vi "HFRR ADV v039.vi"() -> ()   [LabVIEW 2025] (continued)
                      }
                    }
                  }
                }
              }
            }
          }
          frame Enabled {
          }
        }
        n284 = Get Date/Time In Seconds() -> (seconds since 1Jan1904=w369:timestamp)
        n285 = Format Into String(format string="%<%I:%M:%S:%p %d:%B:%Y>T", w369) -> (resulting string=→"Time Stamp":string)  [unwired: 2 in, 1 out]
        n286 = local read "Service Password enable"() -> (w361:bool)
        n287 = local read "FILE"() -> (w366:string)
        n288 = call <vilib>:"Trim Whitespace.vi"("string"=w366) -> ("trimmed string"=w365:string)  [unwired: 1 in]
        n289 = String Length(string=w365) -> (length=w364:i32)
        n290 = Greater?(x=w364, y=1) -> (0:w362:bool)
        n291 = case shown="False" w362 {
          tunnel: w361 -> [w390 _]
          frame False {
            n292 = case shown="False" w390 {
              frame True {
                w391 = "Test Start In Service Mode" ("Tip Strip")
                w392 = T19."Enabled" ("Disabled")
                n293 = property on="Auto Start Test" class="Bool (strict)"("DisabledEnum"=w392, "TipStrip"=w391) -> ()  [unwired: 2 in, 2 out]
                n294 = property on="RUN" class="Bool (strict)"("DisabledEnum"=w392, "TipStrip"=w391) -> ()  [unwired: 2 in, 2 out]
              }
              frame False {
                w393 = "Enter File Name to Start Test" ("Tip Strip")
                w394 = T19."Disabled and Grayed Out" ("Disabled")
                n295 = property on="Auto Start Test" class="Bool (strict)"("DisabledEnum"=w394, "TipStrip"=w393) -> ()  [unwired: 2 in, 2 out]
                n296 = property on="RUN" class="Bool (strict)"("DisabledEnum"=w394, "TipStrip"=w393) -> ()  [unwired: 2 in, 2 out]
              }
            }
          }
          frame True {
            w395 = "" ("Tip Strip")
            w396 = T19."Enabled" ("Disabled")
            n297 = property on="Auto Start Test" class="Bool (strict)"("DisabledEnum"=w396, "TipStrip"=w395) -> ()  [unwired: 2 in, 2 out]
            n298 = property on="RUN" class="Bool (strict)"("DisabledEnum"=w396, "TipStrip"=w395) -> ()  [unwired: 2 in, 2 out]
          }
        }
      }
      event "RUN": Value Change {
        n299 = event-data() -> ()  [unwired: 1 in, 6 out]
        n300 = local read "RUN"() -> (w398:bool)
        n301 = case shown="False" w398 {
          frame False {
            n302 = flat-sequence {
              frame #0 {
                n303 = local write "START TEMP"(FALSE ("START TEMP")) -> ()
              }
              frame #1 {
                n304 = Wait (ms)(milliseconds to wait=u32 1500) -> ()  [unwired: 1 out]
              }
              frame #2 {
                n305 = local write "Humidity 2"(TRUE ("Humidity")) -> ()
              }
              frame #3 {
                n306 = local write "Due Write"("VC;0") -> ()
              }
              frame #4 {
                n307 = Wait (ms)(milliseconds to wait=u32 1500) -> ()  [unwired: 1 out]
              }
              frame #5 {
                w408 = T19."Enabled" ("Disabled")
                (unwired) T26."Imaging" ("Main Dashboard Buttons")
                (unwired) T21."Adv Scar" ("Main Tab")
                w410 = "" ("FILE")
                n308 = local write "measured_stroke"(0.0 ("measured_stroke")) -> ()
                n309 = local write "Due Write"("VC;0") -> ()
                n310 = local write "FILE"(w410) -> ()
                n311 = local write "Batch Ref Num :"(w410) -> ()
                n312 = local write "Fuel Discription :"(w410) -> ()
                n313 = local write "Main Tab"(T2."Adv Scar" ("Main Tab")) -> ()
                n314 = local write "Remarks :"(w410) -> ()
                n315 = local write "Main Dashboard Buttons"(T1."Imaging" ("Main Dashboard Buttons")) -> ()
                n316 = local write "TEST FILE NAM,E SAVED"(FALSE ("TEST FILE NAM,E SAVED")) -> ()
                n317 = property on="Stroke ( mm )" class="WFChart (strict)"("History Data"=cluster{"y":dbl, dbl, "y":dbl}[] []) -> ()  [unwired: 2 in, 2 out]
                n318 = property on="Auto Start Test" class="Bool (strict)"("Visible"=TRUE) -> ()  [unwired: 2 in, 2 out]
                n319 = property on="FRICVALZ 2" class="Bool (strict)"("DisabledEnum"=w408) -> ()  [unwired: 2 in, 2 out]
                n320 = property on="FRICVALZ 4" class="Bool (strict)"("DisabledEnum"=w408) -> ()  [unwired: 2 in, 2 out]
                n321 = property on="FRICVALZ 3" class="Bool (strict)"("DisabledEnum"=w408) -> ()  [unwired: 2 in, 2 out]
              }
            }
          }
          frame True {
            n322 = stacked-sequence {
              frame #0 {
                n323 = local write "Due Write"("DAC;200") -> ()
              }
              frame #1 {
                n324 = Wait (ms)(milliseconds to wait=u32 1500) -> ()  [unwired: 1 out]
              }
              frame #2 {
                n325 = local write "Due Write"("DAC;200") -> ()
              }
              frame #3 {
                n326 = Wait (ms)(milliseconds to wait=u32 1500) -> ()  [unwired: 1 out]
              }
              frame #4 {
                n327 = local write "Due Write"("VC;1") -> ()
              }
              frame #5 {
                n328 = Wait (ms)(milliseconds to wait=u32 2000) -> ()  [unwired: 1 out]
              }
              frame #6 {
                n329 = local write "Due Write"("VC;1") -> ()
              }
              frame #7 {
                n330 = Wait (ms)(milliseconds to wait=u32 2000) -> ()  [unwired: 1 out]
              }
              frame #8 {
                w422 = T19."Disabled" ("Disabled")
                n331 = property on="Auto Start Test" class="Bool (strict)"("Visible"=FALSE) -> ()  [unwired: 2 in, 2 out]
                n332 = local write "START TEMP"(TRUE ("START TEMP")) -> ()
                n333 = property on="FRICVALZ 2" class="Bool (strict)"("DisabledEnum"=w422) -> ()  [unwired: 2 in, 2 out]
                n334 = property on="FRICVALZ 4" class="Bool (strict)"("DisabledEnum"=w422) -> ()  [unwired: 2 in, 2 out]
                n335 = property on="FRICVALZ 3" class="Bool (strict)"("DisabledEnum"=w422) -> ()  [unwired: 2 in, 2 out]
              }
            }
          }
        }
      }
      event "run test Calibration": Value Change {
        n336 = event-data() -> ()  [unwired: 1 in, 6 out]
        n337 = local read "run test Calibration"() -> (w424:bool)
        n338 = case shown="True" w424 {
          frame False {
            n339 = flat-sequence {
              frame #0 {
                n340 = local write "START TEMP"(FALSE ("START TEMP")) -> ()
              }
              frame #1 {
                n341 = Wait (ms)(milliseconds to wait=u32 1500) -> ()  [unwired: 1 out]
              }
              frame #2 {
              }
              frame #3 {
                n342 = local write "Due Write"("VC;0") -> ()
              }
              frame #4 {
                n343 = Wait (ms)(milliseconds to wait=u32 1500) -> ()  [unwired: 1 out]
              }
              frame #5 {
                n344 = local write "Due Write"("VC;0") -> ()
              }
            }
          }
          frame True {
            n345 = flat-sequence {
              frame #0 {
                n346 = local write "Due Write"("VC;1") -> ()
              }
              frame #1 {
                n347 = Wait (ms)(milliseconds to wait=u32 2000) -> ()  [unwired: 1 out]
              }
              frame #2 {
                n348 = local write "Due Write"("VC;1") -> ()
              }
              frame #3 {
                n349 = Wait (ms)(milliseconds to wait=u32 2000) -> ()  [unwired: 1 out]
              }
              frame #4 {
                n350 = local write "START TEMP"(TRUE ("START TEMP")) -> ()
              }
            }
          }
        }
      }
      event "Auto": Value Change {
        n351 = event-data() -> ()  [unwired: 1 in, 6 out]
        n352 = stacked-sequence {
          frame #0 {
            n353 = local write "FILE"("") -> ()
          }
          frame #1 {
            n354 = Get Date/Time In Seconds() -> (seconds since 1Jan1904=w440:timestamp)
            n355 = Format Into String(format string="%<%I_%M_%S_%p_%d_%B_%Y>T", w440) -> (resulting string=w439:string)  [unwired: 2 in, 1 out]
            n356 = local write "FILE"(w439) -> ()
          }
        }
        n357 = local read "Auto"() -> (w437:bool)
        n358 = Not(x=w437) -> (.not. x?=w436:bool)
        n359 = local write "Auto"(w436) -> ()
      }
      event "Auto Start Temp": Value Change {
        n360 = event-data() -> ()  [unwired: 1 in, 6 out]
        n361 = local read "Auto Start Test"() -> (w443:bool)
        n362 = case shown="False" w443 {
          frame False {
            n363 = stacked-sequence {
              frame #0 {
                n364 = local write "START TEMP"(FALSE ("START TEMP")) -> ()
              }
              frame #1 {
                n365 = Wait (ms)(milliseconds to wait=u32 2000) -> ()  [unwired: 1 out]
              }
              frame #2 {
                n366 = local write "Due Write"("VC;0") -> ()
              }
              frame #3 {
                n367 = Wait (ms)(milliseconds to wait=u32 2000) -> ()  [unwired: 1 out]
              }
              frame #4 {
                w454 = T19."Enabled" ("Disabled")
                (unwired) T26."Imaging" ("Main Dashboard Buttons")
                w455 = "" ("FILE")
                n368 = local write "Main Tab"(T2."Adv Scar" ("Main Tab")) -> ()
                n369 = local write "measured_stroke"(0.0 ("measured_stroke")) -> ()
                n370 = local write "Main Dashboard Buttons"(T1."Imaging" ("Main Dashboard Buttons")) -> ()
                n371 = property on="RUN" class="Bool (strict)"("Visible"=TRUE) -> ()  [unwired: 2 in, 2 out]
                n372 = local write "Due Write"("VC;0") -> ()
                n373 = local write "Humidity 2"(TRUE ("Humidity")) -> ()
                n374 = local write "TEST FILE NAM,E SAVED"(FALSE ("TEST FILE NAM,E SAVED")) -> ()
                n375 = local write "Fuel Discription :"(w455) -> ()
                n376 = local write "Batch Ref Num :"(w455) -> ()
                n377 = local write "Remarks :"(w455) -> ()
                n378 = local write "FILE"(w455) -> ()
                n379 = property on="FRICVALZ 2" class="Bool (strict)"("DisabledEnum"=w454) -> ()  [unwired: 2 in, 2 out]
                n380 = property on="FRICVALZ 4" class="Bool (strict)"("DisabledEnum"=w454) -> ()  [unwired: 2 in, 2 out]
                n381 = property on="FRICVALZ 3" class="Bool (strict)"("DisabledEnum"=w454) -> ()  [unwired: 2 in, 2 out]
              }
            }
          }
          frame True {
            n382 = stacked-sequence {
              frame #0 {
                n383 = local write "Due Write"("DAC;200") -> ()
              }
              frame #1 {
                n384 = Wait (ms)(milliseconds to wait=u32 1500) -> ()  [unwired: 1 out]
              }
              frame #2 {
                n385 = local write "Due Write"("DAC;200") -> ()
              }
              frame #3 {
                n386 = Wait (ms)(milliseconds to wait=u32 1000) -> ()  [unwired: 1 out]
              }
              frame #4 {
                n387 = local write "Due Write"("VC;1") -> ()
              }
              frame #5 {
                n388 = Wait (ms)(milliseconds to wait=u32 2000) -> ()  [unwired: 1 out]
              }
              frame #6 {
                n389 = local write "Due Write"("VC;1") -> ()
              }
              frame #7 {
                n390 = Wait (ms)(milliseconds to wait=u32 2000) -> ()  [unwired: 1 out]
              }
              frame #8 {
                w466 = T19."Disabled" ("Disabled")
                n391 = property on="RUN" class="Bool (strict)"("Visible"=FALSE) -> ()  [unwired: 2 in, 2 out]
                n392 = property on="FRICVALZ 2" class="Bool (strict)"("DisabledEnum"=w466) -> ()  [unwired: 2 in, 2 out]
                n393 = property on="FRICVALZ 4" class="Bool (strict)"("DisabledEnum"=w466) -> ()  [unwired: 2 in, 2 out]
                n394 = property on="FRICVALZ 3" class="Bool (strict)"("DisabledEnum"=w466) -> ()  [unwired: 2 in, 2 out]
                "START TEMP" <- TRUE
              }
            }
          }
        }
      }
      event "FILE", "USERNAME", "USER ID": Mouse Enter {
        n395 = event-data() -> ()  [unwired: 1 in, 4 out]
        n396 = dll-call lib="kernel32.dll" fn="Wow64DisableWow64FsRedirection"("OldValue"=0) -> (error out=w473:errorcluster, "OldValue"=w471:i32)  [unwired: 4 in, 1 out]
        n397 = call <vilib>:"System Exec.vi"("run minimized? (F)"=TRUE, "error in (no error)"=w473, "command line"="C:\\Program Files\\Common Files\\Microsoft Shared\\Ink\\TabTip.exe") -> ("error out"=w472:errorcluster)  [unwired: 5 in, 3 out]
        n398 = dll-call lib="kernel32.dll" fn="Wow64EnableWow64FsRedirection"(error in=w472, "OldValue"=w471) -> ()  [unwired: 4 in, 2 out]
      }
      event "EDIT": Value Change {
        n399 = event-data() -> ()  [unwired: 1 in, 6 out]
        n400 = local read "EDIT"() -> (w474:bool)
        n401 = case shown="False" w474 {
          frame False {
            n402 = control-ref of="This VI"() -> (w491:refnum<vi>)
            n403 = property class="VI"(reference=w491) -> (reference out=w482:refnum<vi>, error out=w486:errorcluster, "Panel"=w490:refnum<vi>)  [unwired: 1 in]
            n404 = property class="Pnl"(reference=w490, error in=w486) -> (reference out=w484:refnum<vi>, error out=w487:errorcluster, "Panes[]"=w489:refnum<vi>[])
            n405 = for {
              tunnel: w489 -> [w497] mode=indexing
              tunnel: T24."Always Off" ("Horizontal Scrollbar Visibility") -> [w496]
              tunnel: w487 -> [w493]
              tunnel: [w492] -> w485
              n406 = property class="Pane"(reference=w497, error in=w493, "HorizScrollbarVisibility"=w496) -> (reference out=w494:refnum<vi>, error out=w495:errorcluster)
              n407 = Close Reference(reference=w494, error in (no error)=w495) -> (error out=w492:errorcluster)
            }
            n408 = Close Reference(reference=w484, error in (no error)=w485) -> (error out=w483:errorcluster)
            n409 = Close Reference(reference=w482, error in (no error)=w483) -> (error out=w477:errorcluster)
            "error out 7" <- w477
            n410 = call <vilib>:"Clear Errors.vi"("error in (no error)"=w477) -> ("error out"=w476:errorcluster)  [unwired: 5 in, 1 out]
            n411 = local write "Service Password enable"(FALSE ("Service Password enable")) -> ()
            n412 = call <userlib>:"Fit VI window to Largest Dec.vi"("error in (no error)"=w476, "border spacing (2 px)"=1) -> ("error out"=w481:errorcluster, "dup VI Ref"=w479:refnum<vi>)  [unwired: 4 in]
            n413 = invoke on="Invoke Node" class="VI" method="FP.Run-Time Position.Maximized"(reference=w479, error in=w481) -> (error out=w480:errorcluster)  [unwired: 2 in, 3 out]
            n414 = call <vilib>:"Clear Errors.vi"("error in (no error)"=w480) -> ()  [unwired: 5 in, 2 out]
          }
          frame True {
          }
        }
      }
      event "Heater Button": Value Change {
        n415 = event-data() -> ()  [unwired: 1 in, 6 out]
        n416 = local read "Heater Button"() -> (w498:bool)
        n417 = case shown="True" w498 {
          frame True {
            n418 = stacked-sequence {
              frame #0 {
                n419 = Wait (ms)(milliseconds to wait=u32 1500) -> ()  [unwired: 1 out]
              }
              frame #1 {
                n420 = local read "Set Temp"() -> (w500:dbl)
                n421 = Number To Fractional String(number=w500, precision (6)=i16 2) -> (F-format string=w503:string)  [unwired: 2 in]
                n422 = Concatenate Strings("ST;" ("Command"), w503) -> (w502:string)
                n423 = local write "Due Write"(w502) -> ()
              }
              frame #2 {
                n424 = Wait (ms)(milliseconds to wait=u32 1500) -> ()  [unwired: 1 out]
              }
              frame #3 {
                n425 = local write "Due Write"("HE;1" ("Command")) -> ()
              }
              frame #4 {
                n426 = Wait (ms)(milliseconds to wait=u32 1500) -> ()  [unwired: 1 out]
              }
              frame #5 {
                n427 = stacked-sequence {
                  frame #0 {
                    n428 = Wait (ms)(milliseconds to wait=u32 1500) -> ()  [unwired: 1 out]
                  }
                  frame #1 {
                    n429 = local read "Set Temp"() -> (w509:dbl)
                    n430 = Number To Fractional String(number=w509, precision (6)=i16 2) -> (F-format string=w512:string)  [unwired: 2 in]
                    n431 = Concatenate Strings("ST;" ("Command"), w512) -> (w511:string)
                    n432 = local write "Due Write"(w511) -> ()
                  }
                  frame #2 {
                    n433 = Wait (ms)(milliseconds to wait=u32 1500) -> ()  [unwired: 1 out]
                  }
                  frame #3 {
                    n434 = local write "Due Write"("HE;1" ("Command")) -> ()
                  }
                  frame #4 {
                    n435 = Wait (ms)(milliseconds to wait=u32 1500) -> ()  [unwired: 1 out]
                  }
                }
              }
            }
          }
          frame False {
            n436 = stacked-sequence {
              frame #0 {
                n437 = Wait (ms)(milliseconds to wait=u32 1500) -> ()  [unwired: 1 out]
              }
              frame #1 {
                n438 = Concatenate Strings("ST;" ("Command"), "0" ("string")) -> (w519:string)
                n439 = local write "Due Write"(w519) -> ()
              }
              frame #2 {
                n440 = Wait (ms)(milliseconds to wait=u32 1500) -> ()  [unwired: 1 out]
              }
              frame #3 {
                n441 = local write "Due Write"("HE;0" ("Command")) -> ()
              }
              frame #4 {
                n442 = Wait (ms)(milliseconds to wait=u32 1500) -> ()  [unwired: 1 out]
              }
            }
          }
        }
      }
      event "Headen Service Button": Value Change {
        n443 = event-data() -> ()  [unwired: 1 in, 6 out]
        n444 = local read "Headen Service Button"() -> (w524:bool)
        n445 = case shown="True" w524 {
          frame False {
            n446 = property on="Password 3" class="Clust (strict)"("Visible"=FALSE) -> ()  [unwired: 2 in, 2 out]
            n447 = property on="Service Password Log" class="Str"("Visible"=FALSE) -> ()  [unwired: 2 in, 2 out]
          }
          frame True {
            n448 = property on="Password 3" class="Clust (strict)"("Visible"=TRUE) -> ()  [unwired: 2 in, 2 out]
            n449 = property on="Service Password Log" class="Str"("Visible"=TRUE) -> ()  [unwired: 2 in, 2 out]
          }
        }
      }
      event "Password 3.Service Password": Value Change {
        n450 = event-data() -> ()  [unwired: 1 in, 6 out]
        n451 = Unbundle By Name("Password 3") -> ("Service Password"=w531:string)
        n452 = call <vilib>:"Trim Whitespace.vi"("string"=w531) -> ("trimmed string"=w529:string)  [unwired: 1 in]
        n453 = Equal?(x=w529, y="Service@123") -> (x = y?=w530:bool)
        n454 = case shown="False" w530 {
          selector: w530 -> [w534 w536]
          frame False {
            n455 = local write "Service Password enable"(w534) -> ()
            n456 = property on="Service Password Log" class="Str"("Visible"=TRUE) -> ()  [unwired: 2 in, 2 out]
          }
          frame True {
            n457 = property on="Service Password Log" class="Str"("Visible"=FALSE) -> ()  [unwired: 2 in, 2 out]
            "Service Password enable" <- w536
          }
        }
      }
      event "Sign In": Value Change {
        w538 = FALSE ("Visible")
        n458 = event-data() -> ()  [unwired: 1 in, 6 out]
        n459 = property on="About" class="Clust (strict)"("Visible"=w538) -> ()  [unwired: 2 in, 2 out]
        n460 = property on="Password 3" class="Clust (strict)"("Visible"=w538) -> ()  [unwired: 2 in, 2 out]
        n461 = property on="Service Password Log" class="Str"("Visible"=FALSE) -> ()  [unwired: 2 in, 2 out]
      }
      event "Info": Value Change {
        n462 = event-data() -> ()  [unwired: 1 in, 6 out]
        n463 = local read "Info"() -> (w540:bool)
        n464 = case shown="False" w540 {
          frame False {
            n465 = property on="About" class="Clust (strict)"("Visible"=FALSE) -> ()  [unwired: 2 in, 2 out]
          }
          frame True {
            n466 = property on="About" class="Clust (strict)"("Visible"=TRUE) -> ()  [unwired: 2 in, 2 out]
          }
        }
      }
      event "Calibration": Value Change {
        n467 = event-data() -> ()  [unwired: 1 in, 6 out]
        n468 = local read "Calibration"() -> (w544:bool)
        n469 = case shown="False" w544 {
          frame False {
            n470 = property on="Calibration 2" class="TabCtl (strict)"("Visible"=FALSE) -> ()  [unwired: 2 in, 2 out]
            n471 = local write "Cal Password"("" ("Cal Password")) -> ()
          }
          frame True {
            n472 = property on="Calibration 2" class="TabCtl (strict)"("Visible"=TRUE) -> ()  [unwired: 2 in, 2 out]
            n473 = local write "Cal Password"("" ("Cal Password")) -> ()
          }
        }
        n474 = property on="Wrong Password" class="Str"("Visible"=FALSE) -> ()  [unwired: 2 in, 2 out]
      }
      event "Cal Password": Value Change {
        n475 = event-data() -> ()  [unwired: 1 in, 6 out]
        n476 = local read "Cal Password"() -> (w552:string)
        n477 = call <vilib>:"Trim Whitespace.vi"("string"=w552) -> ("trimmed string"=w551:string)  [unwired: 1 in]
        n478 = Equal?(x=w551, y="Cal@321") -> (x = y?=w549:bool)
        n479 = case shown="True" w549 {
          frame False {
            n480 = property on="Wrong Password" class="Str"("Visible"=TRUE) -> ()  [unwired: 2 in, 2 out]
          }
          frame True {
            n481 = property on="Wrong Password" class="Str"("Visible"=FALSE) -> ()  [unwired: 2 in, 2 out]
            n482 = local write "Main Tab"(T2."About" ("Main Tab")) -> ()
            n483 = local write "Cal Password"("" ("Cal Password")) -> ()
            n484 = local write "Main Dashboard Buttons"(T1."About" ("Main Dashboard Buttons")) -> ()
            n485 = property on="Calibration 2" class="TabCtl (strict)"("Visible"=FALSE) -> ()  [unwired: 2 in, 2 out]
            n486 = local write "Calibration"(FALSE ("Calibration")) -> ()
          }
        }
      }
      event "Calibration Selection": Value Change {
        n487 = event-data() -> ()  [unwired: 1 in, 6 out]
        n488 = local read "Calibration Selection"() -> (w561:T8)
        n489 = case shown="\"Stroke Calibration\"" w561 {
          tunnel: [T7."Stroke" ("Main Calibration Tab") T7."Friction" ("Main Calibration Tab") T7."Main" ("Main Calibration Tab") T7."Temperature" ("Main Calibration Tab")] -> w560
          frame "Stroke Calibration" {
          }
          frame "Friction Force Calibration" {
          }
          frame Default {
          }
          frame "Temperature Calibration" {
          }
        }
        n490 = local write "Main Calibration Tab"(w560) -> ()
      }
      event "Back Stroke": Value Change {
        n491 = event-data() -> ()  [unwired: 1 in, 6 out]
        n492 = local write "Main Stroke Tab"(T9."Step 1" ("Main Stroke Tab")) -> ()
        n493 = local write "Main Calibration Tab"(T7."Main" ("Main Calibration Tab")) -> ()
        n494 = local write "Back Stroke"(FALSE ("Back Stroke")) -> ()
      }
      event "Step 2 Back": Value Change {
        n495 = event-data() -> ()  [unwired: 1 in, 6 out]
        n496 = local write "Main Stroke Tab"(T9."Step 1" ("Main Stroke Tab")) -> ()
        n497 = local write "Step 2 Back"(FALSE ("Back Stroke")) -> ()
      }
      event "Step 3 Back": Value Change {
        n498 = event-data() -> ()  [unwired: 1 in, 6 out]
        n499 = local write "Main Stroke Tab"(T9."Step 2" ("Main Stroke Tab")) -> ()
        n500 = local write "Step 3 Back"(FALSE ("Back Stroke")) -> ()
      }
      event "Step 4 Back": Value Change {
        n501 = event-data() -> ()  [unwired: 1 in, 6 out]
        n502 = local write "Main Stroke Tab"(T9."Step 3" ("Main Stroke Tab")) -> ()
        n503 = local write "Step 4 Back"(FALSE ("Back Stroke")) -> ()
      }
      event "Step 5 Back": Value Change {
        n504 = event-data() -> ()  [unwired: 1 in, 6 out]
        n505 = local write "Main Stroke Tab"(T9."Step 4" ("Main Stroke Tab")) -> ()
        n506 = local write "Step 5 Back"(FALSE ("Back Stroke")) -> ()
      }
      event "Step 6 Back": Value Change {
        n507 = event-data() -> ()  [unwired: 1 in, 6 out]
        n508 = local write "Main Stroke Tab"(T9."Step 5" ("Main Stroke Tab")) -> ()
        n509 = local write "Step 6 Back"(FALSE ("Back Stroke")) -> ()
      }
      event "Back Stroke step 7": Value Change {
        n510 = event-data() -> ()  [unwired: 1 in, 6 out]
        n511 = local write "Main Stroke Tab"(T9."Step 5" ("Main Stroke Tab")) -> ()
        n512 = local write "Back Stroke step 7"(FALSE ("Back Stroke")) -> ()
      }
      event "Back Stroke step 8": Value Change {
        n513 = event-data() -> ()  [unwired: 1 in, 6 out]
        n514 = local write "Main Stroke Tab"(T9."Step 7" ("Main Stroke Tab")) -> ()
        n515 = local write "Back Stroke step 8"(FALSE ("Back Stroke")) -> ()
      }
      event "Back Stroke 8": Value Change {
        n516 = event-data() -> ()  [unwired: 1 in, 6 out]
        n517 = local write "MOVE CARRIAGE TO"(0.2 ("MOVE CARRIAGE TO")) -> ()
        n518 = local write "Main Stroke Tab"(T9."Step 1" ("Main Stroke Tab")) -> ()
        n519 = local write "Back Stroke 8"(FALSE ("Back Stroke 8")) -> ()
      }
      event "Continue Stroke": Value Change {
        n520 = event-data() -> ()  [unwired: 1 in, 6 out]
        n521 = local write "Main Stroke Tab"(T9."Step 2" ("Main Stroke Tab")) -> ()
        n522 = local write "Continue Stroke"(FALSE ("Continue Stroke")) -> ()
      }
      event "Continue Stroke step 2": Value Change {
        n523 = event-data() -> ()  [unwired: 1 in, 6 out]
        n524 = local write "Main Stroke Tab"(T9."Step 3" ("Main Stroke Tab")) -> ()
        n525 = local write "Continue Stroke step 2"(FALSE ("Continue Stroke")) -> ()
      }
      event "Continue Stroke step 3": Value Change {
        n526 = event-data() -> ()  [unwired: 1 in, 6 out]
        n527 = local write "Main Stroke Tab"(T9."Step 4" ("Main Stroke Tab")) -> ()
        n528 = local write "Continue Stroke step 3"(FALSE ("Continue Stroke")) -> ()
      }
      event "Continue Stroke step 4": Value Change {
        n529 = event-data() -> ()  [unwired: 1 in, 6 out]
        n530 = local write "Main Stroke Tab"(T9."Step 5" ("Main Stroke Tab")) -> ()
        n531 = local write "Continue Stroke step 4"(FALSE ("Continue Stroke")) -> ()
      }
      event "Continue Stroke step 5": Value Change {
        n532 = event-data() -> ()  [unwired: 1 in, 6 out]
        n533 = local write "Main Stroke Tab"(T9."Step 7" ("Main Stroke Tab")) -> ()
        n534 = local write "Continue Stroke step 5"(FALSE ("Continue Stroke")) -> ()
      }
      event "Continue Stroke step 6": Value Change {
        n535 = event-data() -> ()  [unwired: 1 in, 6 out]
        n536 = local write "Main Stroke Tab"(T9."Step 7" ("Main Stroke Tab")) -> ()
        n537 = local write "Continue Stroke step 6"(FALSE ("Continue Stroke")) -> ()
      }
      event "Continue Stroke step 7": Value Change {
        w600 = FALSE ("0.2mm")
        n538 = event-data() -> ()  [unwired: 1 in, 6 out]
        n539 = local write "0.4 mm"(w600) -> ()
        n540 = local write "0.6 mm"(w600) -> ()
        n541 = local write "1.0 mm"(w600) -> ()
        n542 = local write "1.2 mm"(w600) -> ()
        n543 = local write "0.2 2"(w600) -> ()
        n544 = local write "0.4 2"(w600) -> ()
        n545 = local write "0.6 2"(w600) -> ()
        n546 = local write "0.8 2"(w600) -> ()
        n547 = local write "1.0 2"(w600) -> ()
        n548 = local write "1.2"(w600) -> ()
        n549 = local write "0.2mm"(w600) -> ()
        n550 = local write "0.8mm"(w600) -> ()
        n551 = local write "Main Stroke Tab"(T9."Step 8" ("Main Stroke Tab")) -> ()
        n552 = local write "Continue Stroke step 7"(FALSE ("Continue Stroke")) -> ()
        n553 = local write "Stroke Test Complete"(T10."Test Progress" ("Stroke Test Complete")) -> ()
        "Position Measurment Temp" <- 4.0 ("Position Measurment Temp")
        "Calibration Tare" <- TRUE ("Calibration Tare")
        "MOVE CARRIAGE TO" <- 1.0 ("MOVE CARRIAGE TO")
      }
      event "Continue Stroke step 8": Value Change {
        n554 = event-data() -> ()  [unwired: 1 in, 6 out]
        n555 = local read "LVDT STROKE  Calibration"() -> (w605:dbl)
        n556 = local read "Position Measurment Temp"() -> (w606:dbl)
        n557 = case shown="0, Default" w606 {
          selector: w606 -> [w611 w616 w621 w626 _ w634 w637 w638]
          tunnel: w605 -> [w607 w612 w617 w622 w628 w631 _ _]
          frame 0, Default {
            w609 = TRUE ("0.2mm")
            n558 = Increment(x=w611) -> (x+1=w610:i32)
            n559 = local write "Position Measurment Temp"(w610) -> ()
            n560 = local write "0.2mm"(w609) -> ()
            n561 = local write "0.2 2"(w609) -> ()
            n562 = local write "MOVE CARRIAGE TO"(1.0 ("MOVE CARRIAGE TO")) -> ()
            "Calibration 0.2" <- w607
          }
          frame 1 {
            w614 = TRUE ("0.4 mm")
            n563 = Increment(x=w616) -> (x+1=w615:i32)
            n564 = local write "Calibration 0.4"(w612) -> ()
            n565 = local write "Position Measurment Temp"(w615) -> ()
            n566 = local write "0.4 mm"(w614) -> ()
            n567 = local write "MOVE CARRIAGE TO"(0.6 ("MOVE CARRIAGE TO")) -> ()
            n568 = local write "0.4 2"(w614) -> ()
          }
          frame 2 {
            w619 = TRUE ("0.6 mm")
            n569 = Increment(x=w621) -> (x+1=w620:i32)
            n570 = local write "Calibration 0.6"(w617) -> ()
            n571 = local write "Position Measurment Temp"(w620) -> ()
            n572 = local write "0.6 2"(w619) -> ()
            n573 = local write "0.6 mm"(w619) -> ()
            n574 = local write "MOVE CARRIAGE TO"(0.8 ("MOVE CARRIAGE TO")) -> ()
          }
          frame 3 {
            w623 = TRUE ("0.6 mm")
            n575 = Increment(x=w626) -> (x+1=w625:i32)
            n576 = local write "Position Measurment Temp"(w625) -> ()
            n577 = local write "MOVE CARRIAGE TO"(1.0 ("MOVE CARRIAGE TO")) -> ()
            n578 = local write "0.8mm"(w623) -> ()
            n579 = local write "0.8 2"(w623) -> ()
            "Calibration 0.8" <- w622
          }
          frame 4 {
            w629 = TRUE ("0.6 mm")
            n580 = local write "Position Measurment Temp"(6.0 ("Position Measurment Temp")) -> ()
            n581 = local write "MOVE CARRIAGE TO"(1.0 ("MOVE CARRIAGE TO")) -> ()
            n582 = local write "1.0 mm"(w629) -> ()
            n583 = local write "1.0 2"(w629) -> ()
            "Calibration 1.0" <- w628
          }
          frame 5 {
            w632 = TRUE ("0.6 mm")
            n584 = Increment(x=w634) -> (x+1=w633:i32)
            n585 = local write "Position Measurment Temp"(w633) -> ()
            n586 = local write "1.2 mm"(w632) -> ()
            n587 = local write "1.2"(w632) -> ()
            "Calibration 1.2" <- w631
          }
          frame 6 {
            n588 = Increment(x=w637) -> (x+1=w636:i32)
            n589 = local write "Position Measurment Temp"(w636) -> ()
            n590 = local write "Stroke Test Complete"(T10."Stroke Points Completed" ("Stroke Test Complete")) -> ()
          }
          frame 7 {
            n591 = stacked-sequence {
              tunnel: w638 -> [w639 _ _]
              frame #0 {
                n592 = Increment(x=w639) -> (x+1=w640:i32)
                n593 = local write "Main Stroke Tab"(T9."Step 9" ("Main Stroke Tab")) -> ()
                n594 = local write "Position Measurment Temp"(w640) -> ()
                n595 = Insert Into Array(array=dbl[] [], new element #1=0.2 ("new element/subarray"), new element #2=0.4 ("new element/subarray"), new element #3=0.6 ("new element/subarray"), new element #4=0.8 ("new element/subarray"), new element #5=1.0 ("new element/subarray"), new element #6=1.2 ("new element/subarray")) -> (→"1D stroke":dbl[])  [unwired: 1 in]
                n596 = local read "Calibration 0.2"() -> (w647:dbl)
                n597 = local read "Calibration 0.4"() -> (w646:dbl)
                n598 = local read "Calibration 0.6"() -> (w645:dbl)
                n599 = local read "Calibration 0.8"() -> (w644:dbl)
                n600 = local read "Calibration 1.0"() -> (w643:dbl)
                n601 = local read "Calibration 1.2"() -> (w642:dbl)
                n602 = Insert Into Array(array=dbl[] [], new element #1=w647, new element #2=w646, new element #3=w645, new element #4=w644, new element #5=w643, new element #6=w642) -> (→"Calibrated Voltage Value":dbl[])  [unwired: 1 in]
              }
              frame #1 {
                n603 = local read "calibration values"() -> (w670:dbl[])
                n604 = local read "Calibrated Voltage Value"() -> (w672:dbl[])
                n605 = Index Array(array=w670, index #1=1 ("index"), index #2=3 ("index"), index #3=5 ("index"), index #4=7 ("index"), index #5=9 ("index"), index #6=11 ("index")) -> (element #1=w663:dbl, element #2=w662:dbl, element #3=w661:dbl, element #4=w660:dbl, element #5=w659:dbl, element #6=w658:dbl)
                n606 = local read "1D stroke"() -> (w673:dbl[])
                n607 = for {
                  tunnel: [w682] -> w671 mode=indexing
                  tunnel: w673 -> [w681] mode=indexing
                  tunnel: w672 -> [w680] mode=indexing
                  tunnel: w663 -> [w679]
                  tunnel: w662 -> [w678]
                  tunnel: w661 -> [w677]
                  tunnel: w660 -> [w676]
                  tunnel: w659 -> [w675]
                  tunnel: w658 -> [w674]
                  n608 = formula code="if (stroke == 0.2)\n{\n    if ((voltage >= REF_02 - 0.2) && (voltage <= REF_02 + 0.2))\n        status = 1;\n    else\n        status = 0;\n}\nelse if (stroke == 0.4)\n{\n    if ((voltage >= REF_04 - 0.2) && (voltage <= REF_04 + 0.2))\n        status = 1;\n    else\n        status = 0;\n}\nelse if (stroke == 0.6)\n{\n    if ((voltage >= REF_06 - 0.2) && (voltage <= REF_06 + 0.2))\n        status = 1;\n    else\n        status = 0;\n}\nelse if (stroke == 0.8)\n{\n    if ((voltage >= REF_08 - 0.2) && (voltage <= REF_08 + 0.2))\n        status = 1;\n    else\n        status = 0;\n}\nelse if (stroke == 1.0)\n{\n    if ((voltage >= REF_10 - 0.4) && (voltage <= REF_10 + 0.4))\n        status = 1;\n    else\n        status = 0;\n}\nelse if (stroke == 1.2)\n{\n    if ((voltage >= REF_12 - 0.2) && (voltage <= REF_12 + 0.2))\n        status = 1;\n    else\n        status = 0;\n}\nelse\n{\n    status = 0;\n}"("stroke"=w681, "voltage"=w680, "REF_02"=w679, "REF_04"=w678, "REF_06"=w677, "REF_08"=w676, "REF_10"=w675, "REF_12"=w674) -> ("status"=w682:dbl)
                }
                "Status" <- w671
              }
              frame #2 {
                w689 = 1.0
                n609 = local read "Status"() -> (w696:dbl[])
                n610 = Index Array(array=w696) -> (element #1=w695:dbl, element #2=w694:dbl, element #3=w693:dbl, element #4=w692:dbl, element #5=w691:dbl, element #6=w690:dbl)  [unwired: 6 in]
                n611 = Equal?(x=w694, y=w689) -> (x = y?=w687:bool)
                n612 = Equal?(x=w693, y=w689) -> (x = y?=w686:bool)
                n613 = Equal?(x=w692, y=w689) -> (x = y?=w685:bool)
                n614 = Equal?(x=w691, y=w689) -> (x = y?=w684:bool)
                n615 = Equal?(x=w690, y=w689) -> (x = y?=w683:bool)
                n616 = Equal?(x=w695, y=w689) -> (x = y?=w688:bool)
                n617 = case shown="True" w688 {
                  selector: w688 -> [w707 w708]
                  frame True {
                    n618 = local write "Point 1 - 0.2 mm"(w707) -> ()
                    n619 = property on="Point 1 - 0.2 mm" class="Bool"("Caption.Visible"=w707) -> ()  [unwired: 2 in, 2 out]
                  }
                  frame False {
                    n620 = local write "Point 1 - 0.2 mm"(w708) -> ()
                    n621 = property on="Point 1 - 0.2 mm" class="Bool"("Caption.Visible"=w708) -> ()  [unwired: 2 in, 2 out]
                  }
                }
                n622 = case shown="True" w687 {
                  selector: w687 -> [w705 w706]
                  frame True {
                    n623 = local write "Point 2 - 0.4 mm"(w705) -> ()
                    n624 = property on="Point 2 - 0.4 mm" class="Bool"("Caption.Visible"=w705) -> ()  [unwired: 2 in, 2 out]
                  }
                  frame False {
                    n625 = local write "Point 2 - 0.4 mm"(w706) -> ()
                    n626 = property on="Point 2 - 0.4 mm" class="Bool"("Caption.Visible"=w706) -> ()  [unwired: 2 in, 2 out]
                  }
                }
                n627 = case shown="True" w684 {
                  selector: w684 -> [w699 w700]
                  frame True {
                    n628 = local write "Point 5 - 1.0 mm"(w699) -> ()
                    n629 = property on="Point 5 - 1.0 mm" class="Bool"("Caption.Visible"=w699) -> ()  [unwired: 2 in, 2 out]
                  }
                  frame False {
                    n630 = local write "Point 5 - 1.0 mm"(w700) -> ()
                    n631 = property on="Point 5 - 1.0 mm" class="Bool"("Caption.Visible"=w700) -> ()  [unwired: 2 in, 2 out]
                  }
                }
                n632 = case shown="True" w686 {
                  selector: w686 -> [w703 w704]
                  frame True {
                    n633 = local write "Point 3 - 0.6 mm"(w703) -> ()
                    n634 = property on="Point 3 - 0.6 mm" class="Bool"("Caption.Visible"=w703) -> ()  [unwired: 2 in, 2 out]
                  }
                  frame False {
                    n635 = local write "Point 3 - 0.6 mm"(w704) -> ()
                    n636 = property on="Point 3 - 0.6 mm" class="Bool"("Caption.Visible"=w704) -> ()  [unwired: 2 in, 2 out]
                  }
                }
                n637 = case shown="True" w685 {
                  selector: w685 -> [w701 w702]
                  frame True {
                    n638 = local write "Point 4 - 0.8 mm"(w701) -> ()
                    n639 = property on="Point 4 - 0.8 mm" class="Bool"("Caption.Visible"=w701) -> ()  [unwired: 2 in, 2 out]
                  }
                  frame False {
                    n640 = local write "Point 4 - 0.8 mm"(w702) -> ()
                    n641 = property on="Point 4 - 0.8 mm" class="Bool"("Caption.Visible"=w702) -> ()  [unwired: 2 in, 2 out]
                  }
                }
                n642 = case shown="True" w683 {
                  selector: w683 -> [w697 w698]
                  frame True {
                    n643 = local write "Point 6 - 1.2 mm"(w697) -> ()
                    n644 = property on="Point 6 - 1.2 mm" class="Bool"("Caption.Visible"=w697) -> ()  [unwired: 2 in, 2 out]
                  }
                  frame False {
                    n645 = local write "Point 6 - 1.2 mm"(w698) -> ()
                    n646 = property on="Point 6 - 1.2 mm" class="Bool"("Caption.Visible"=w698) -> ()  [unwired: 2 in, 2 out]
                  }
                }
              }
            }
          }
        }
      }
      event "TEMPERATURE STEP Back 1", "TEMPERATURE STEP Back air Temp": Value Change {
        n647 = event-data() -> ()  [unwired: 1 in, 6 out]
        n648 = stacked-sequence {
          frame #0 {
            n649 = local write "Main Calibration Tab"(T7."Main" ("Main Calibration Tab")) -> ()
          }
          frame #1 {
            n650 = Wait (ms)(milliseconds to wait=u32 1000) -> ()  [unwired: 1 out]
          }
          frame #2 {
            n651 = local write "Due Write"("CAL;END" ("Command")) -> ()
          }
          frame #3 {
            n652 = Wait (ms)(milliseconds to wait=u32 2000) -> ()  [unwired: 1 out]
          }
          frame #4 {
            n653 = local write "Due Write"("CAL;END" ("Command")) -> ()
          }
        }
      }
      event "Temperature Continue Step 1": Value Change {
        n654 = event-data() -> ()  [unwired: 1 in, 6 out]
        n655 = stacked-sequence {
          frame #0 {
            n656 = Wait (ms)(milliseconds to wait=u32 1500) -> ()  [unwired: 1 out]
          }
          frame #1 {
            n657 = local write "Due Write"("CAL;START" ("Command")) -> ()
          }
          frame #2 {
            n658 = Wait (ms)(milliseconds to wait=u32 1500) -> ()  [unwired: 1 out]
          }
          frame #3 {
            n659 = local write "Due Write"("CAL;START" ("Command")) -> ()
          }
          frame #4 {
            n660 = Wait (ms)(milliseconds to wait=u32 2000) -> ()  [unwired: 1 out]
          }
          frame #5 {
          }
          frame #6 {
            n661 = Wait (ms)(milliseconds to wait=u32 2000) -> ()  [unwired: 1 out]
          }
          frame #7 {
            # "CAL;A1;<true_T>"
            n662 = local write "Due Write"("CAL;A1;0" ("Command")) -> ()
          }
          frame #8 {
            n663 = local write "Tab Control 4"(T12."Step 2" ("Tab Control 4")) -> ()
          }
        }
      }
      event "Temperature Continue Step air Step 1": Value Change {
        n664 = event-data() -> ()  [unwired: 1 in, 6 out]
        n665 = stacked-sequence {
          frame #0 {
            n666 = Wait (ms)(milliseconds to wait=u32 1500) -> ()  [unwired: 1 out]
          }
          frame #1 {
            n667 = local write "Due Write"("CAL;START" ("Command")) -> ()
          }
          frame #2 {
            n668 = Wait (ms)(milliseconds to wait=u32 1500) -> ()  [unwired: 1 out]
          }
          frame #3 {
            n669 = local write "Due Write"("CAL;START" ("Command")) -> ()
          }
          frame #4 {
            n670 = Wait (ms)(milliseconds to wait=u32 2000) -> ()  [unwired: 1 out]
          }
          frame #5 {
          }
          frame #6 {
            n671 = Wait (ms)(milliseconds to wait=u32 2000) -> ()  [unwired: 1 out]
          }
          frame #7 {
            # "CAL;A1;<true_T>"
            n672 = local write "Due Write"("CAL;A1;0" ("Command")) -> ()
          }
          frame #8 {
            n673 = local write "Tab Control 4"(T12."Air Step 2" ("Tab Control 4")) -> ()
          }
        }
      }
      event "Temperature Selection": Value Change {
        n674 = event-data() -> ()  [unwired: 1 in, 6 out]
        n675 = local read "Temperature Selection"() -> (w730:T13)
        n676 = case shown="\"Sample Temperature\"" w730 {
          frame "Air Temperature" {
            n677 = local write "Tab Control 4"(T12."Air Step 1" ("Tab Control 4")) -> ()
          }
          frame "Sample Temperature" {
            n678 = local write "Tab Control 4"(T12."Step 1" ("Tab Control 4")) -> ()
          }
          frame "Default", Default {
          }
        }
      }
      event "Temperature Continue Step 2": Value Change {
        n679 = event-data() -> ()  [unwired: 1 in, 6 out]
        n680 = stacked-sequence {
          frame #0 {
            n681 = stacked-sequence {
              frame #0 {
                n682 = Wait (ms)(milliseconds to wait=u32 1500) -> ()  [unwired: 1 out]
              }
              frame #1 {
                # "CAL;A1;<true_T>"
                n683 = local read "Sensor value"() -> (→"Sample 0deg temp":dbl)
                n684 = local write "Due Write"("CAL;A1;0" ("Command")) -> ()
              }
              frame #2 {
                n685 = Wait (ms)(milliseconds to wait=u32 1500) -> ()  [unwired: 1 out]
              }
              frame #3 {
                # "CAL;A1;<true_T>"
                n686 = local write "Due Write"("CAL;A1;0" ("Command")) -> ()
              }
              frame #4 {
              }
            }
          }
          frame #1 {
            n687 = local write "Tab Control 4"(T12."Step 3" ("Tab Control 4")) -> ()
          }
        }
      }
      event "Temperature Continue Air Step 2": Value Change {
        n688 = event-data() -> ()  [unwired: 1 in, 6 out]
        n689 = stacked-sequence {
          frame #0 {
            n690 = stacked-sequence {
              frame #0 {
                n691 = Wait (ms)(milliseconds to wait=u32 1000) -> ()  [unwired: 1 out]
              }
              frame #1 {
                # "CAL;A1;<true_T>"
                n692 = local write "Due Write"("CAL;A1;0" ("Command")) -> ()
              }
              frame #2 {
                n693 = Wait (ms)(milliseconds to wait=u32 1000) -> ()  [unwired: 1 out]
              }
              frame #3 {
                # "CAL;A1;<true_T>"
                n694 = local write "Due Write"("CAL;A1;0" ("Command")) -> ()
              }
              frame #4 {
                n695 = local read "Sensor value"() -> (→"Air 0deg temp":dbl)
              }
            }
          }
          frame #1 {
            n696 = local write "Tab Control 4"(T12."Air Step 3" ("Tab Control 4")) -> ()
          }
        }
      }
      event "Temperature Continue Step 3": Value Change {
        n697 = event-data() -> ()  [unwired: 1 in, 6 out]
        n698 = stacked-sequence {
          frame #0 {
            n699 = stacked-sequence {
              frame #0 {
                n700 = Wait (ms)(milliseconds to wait=u32 1500) -> ()  [unwired: 1 out]
              }
              frame #1 {
              }
              frame #2 {
              }
              frame #3 {
                # "CAL;A1;<true_T>"
                n701 = local write "Due Write"("CAL;A1;60" ("Command")) -> ()
              }
              frame #4 {
                n702 = Wait (ms)(milliseconds to wait=u32 1000) -> ()  [unwired: 1 out]
              }
              frame #5 {
                # "CAL;A1;<true_T>"
                n703 = local read "Sensor value"() -> (→"Sample 60deg temp":dbl)
                n704 = local write "Due Write"("CAL;A1;60" ("Command")) -> ()
              }
            }
          }
          frame #1 {
            n705 = local read "Sample 0deg temp"() -> (w759:dbl)
            n706 = local read "Sample 60deg temp"() -> (w758:dbl)
            n707 = Add(x=w758, y="Temperature diff") -> (x+y=w756:dbl)
            n708 = Subtract(x=w758, y="Temperature diff") -> (x-y=w755:dbl)
            n709 = Add(x=w759, y="Temperature diff") -> (x+y=w754:dbl)
            n710 = Subtract(x=w759, y="Temperature diff") -> (x-y=w753:dbl)
            n711 = In Range and Coerce(upper limit=w756, x=w758, lower limit=w755) -> (In Range?=w752:bool)  [unwired: 1 out]
            n712 = In Range and Coerce(upper limit=w754, x=w759, lower limit=w753) -> (In Range?=w751:bool)  [unwired: 1 out]
            n713 = And(x=w752, y=w751) -> (x .and. y?=w750:bool)
            n714 = case shown="True" w750 {
              frame False {
                n715 = property on="Accept & Save sample Temperature step 4" class="Bool (strict)"("DisabledEnum"=T19."Disabled" ("Disabled")) -> ()  [unwired: 2 in, 2 out]
                n716 = local write "Sample Temperature Calibration  2"(enum32{"True", "Fail"}."Fail" ("Sample Temperature Calibration  2")) -> ()
              }
              frame True {
                n717 = property on="Accept & Save sample Temperature step 4" class="Bool (strict)"("DisabledEnum"=T19."Enabled" ("Disabled")) -> ()  [unwired: 2 in, 2 out]
                n718 = local write "Sample Temperature Calibration  2"(enum32{"True", "Fail"}."True" ("Sample Temperature Calibration  2")) -> ()
              }
            }
          }
          frame #2 {
          }
          frame #3 {
          }
          frame #4 {
          }
          frame #5 {
          }
          frame #6 {
            # "CAL;END"
          }
          frame #7 {
          }
          frame #8 {
            # "CAL;END"
          }
          frame #9 {
            n719 = local write "Tab Control 4"(T12."Step 4" ("Tab Control 4")) -> ()
          }
        }
      }
      event "Accept & Save sample Temperature step 4": Value Change {
        n720 = event-data() -> ()  [unwired: 1 in, 6 out]
        n721 = stacked-sequence {
          frame #0 {
            n722 = local write "Due Write"("CAL;SAVE" ("Command")) -> ()
          }
          frame #1 {
            n723 = Wait (ms)(milliseconds to wait=u32 1000) -> ()  [unwired: 1 out]
          }
          frame #2 {
            n724 = local write "Due Write"("CAL;SAVE" ("Command")) -> ()
          }
          frame #3 {
            n725 = Wait (ms)(milliseconds to wait=u32 1000) -> ()  [unwired: 1 out]
          }
          frame #4 {
            n726 = local write "Due Write"("CAL;END" ("Command")) -> ()
          }
          frame #5 {
            n727 = Wait (ms)(milliseconds to wait=u32 1000) -> ()  [unwired: 1 out]
          }
          frame #6 {
            n728 = local write "Due Write"("CAL;END" ("Command")) -> ()
            n729 = local write "Tab Control 4"(T12."Main" ("Tab Control 4")) -> ()
            n730 = local write "Main Calibration Tab"(T7."Temperature" ("Main Calibration Tab")) -> ()
          }
        }
      }
      event "Accept & Save Air Temperature step 4": Value Change {
        n731 = event-data() -> ()  [unwired: 1 in, 6 out]
        n732 = stacked-sequence {
          frame #0 {
            n733 = local write "Due Write"("CAL;SAVE" ("Command")) -> ()
          }
          frame #1 {
            n734 = Wait (ms)(milliseconds to wait=u32 1000) -> ()  [unwired: 1 out]
          }
          frame #2 {
            n735 = local write "Due Write"("CAL;SAVE" ("Command")) -> ()
          }
          frame #3 {
            n736 = Wait (ms)(milliseconds to wait=u32 1000) -> ()  [unwired: 1 out]
          }
          frame #4 {
            n737 = local write "Due Write"("CAL;END" ("Command")) -> ()
          }
          frame #5 {
            n738 = Wait (ms)(milliseconds to wait=u32 1000) -> ()  [unwired: 1 out]
          }
          frame #6 {
            n739 = local write "Due Write"("CAL;END" ("Command")) -> ()
            n740 = local write "Tab Control 4"(T12."Main" ("Tab Control 4")) -> ()
            n741 = local write "Main Calibration Tab"(T7."Temperature" ("Main Calibration Tab")) -> ()
          }
        }
      }
      event "Temperature Continue Step 6": Value Change {
        n742 = event-data() -> ()  [unwired: 1 in, 6 out]
        n743 = stacked-sequence {
          frame #0 {
            n744 = stacked-sequence {
              frame #0 {
                n745 = Wait (ms)(milliseconds to wait=u32 1000) -> ()  [unwired: 1 out]
              }
              frame #1 {
              }
              frame #2 {
              }
              frame #3 {
                # "CAL;A1;<true_T>"
                n746 = local write "Due Write"("CAL;A1;60" ("Command")) -> ()
              }
              frame #4 {
                n747 = Wait (ms)(milliseconds to wait=u32 1000) -> ()  [unwired: 1 out]
              }
              frame #5 {
                # "CAL;A1;<true_T>"
                n748 = local write "Due Write"("CAL;A1;60" ("Command")) -> ()
              }
            }
          }
          frame #1 {
            n749 = local read "Sensor value"() -> (→"Air 60deg temp":dbl)
          }
          frame #2 {
          }
          frame #3 {
          }
          frame #4 {
          }
          frame #5 {
          }
          frame #6 {
            # "CAL;END"
          }
          frame #7 {
            n750 = local read "Temperature diff"() -> (w790:dbl)
            n751 = local read "Air 60deg temp"() -> (w789:dbl)
            n752 = local read "Air 0deg temp"() -> (w788:dbl)
            n753 = Add(x=w789, y=w790) -> (x+y=w797:dbl)
            n754 = Subtract(x=w789, y=w790) -> (x-y=w796:dbl)
            n755 = Add(x=w788, y=w790) -> (x+y=w795:dbl)
            n756 = Subtract(x=w788, y=w790) -> (x-y=w794:dbl)
            n757 = In Range and Coerce(upper limit=w797, x=w789, lower limit=w796) -> (In Range?=w793:bool)  [unwired: 1 out]
            n758 = In Range and Coerce(upper limit=w795, x=w788, lower limit=w794) -> (In Range?=w792:bool)  [unwired: 1 out]
            n759 = And(x=w793, y=w792) -> (x .and. y?=w791:bool)
            n760 = case shown="True" w791 {
              frame False {
                n761 = property on="Accept & Save Air Temperature step 4" class="Bool (strict)"("DisabledEnum"=T19."Disabled" ("Disabled")) -> ()  [unwired: 2 in, 2 out]
                n762 = local write "Sample Temperature Calibration"(enum32{"True", "Fail"}."Fail" ("Sample Temperature Calibration  2")) -> ()
              }
              frame True {
                n763 = local write "Sample Temperature Calibration"(enum32{"True", "Fail"}."True" ("Sample Temperature Calibration  2")) -> ()
                n764 = property on="Accept & Save Air Temperature step 4" class="Bool (strict)"("DisabledEnum"=T19."Enabled" ("Disabled")) -> ()  [unwired: 2 in, 2 out]
              }
            }
          }
          frame #8 {
            # "CAL;END"
          }
          frame #9 {
            n765 = local write "Tab Control 4"(T12."Air Step 4" ("Tab Control 4")) -> ()
          }
        }
      }
      event "Back Stroke step main temperature": Value Change {
        n766 = event-data() -> ()  [unwired: 1 in, 6 out]
        n767 = stacked-sequence {
          frame #0 {
            n768 = Wait (ms)(milliseconds to wait=u32 1000) -> ()  [unwired: 1 out]
          }
          frame #1 {
            # "CAL;END"
            n769 = local write "Due Write"("CAL;END" ("Command")) -> ()
          }
          frame #2 {
            n770 = Wait (ms)(milliseconds to wait=u32 1000) -> ()  [unwired: 1 out]
          }
          frame #3 {
            # "CAL;END"
            n771 = local write "Due Write"("CAL;END" ("Command")) -> ()
          }
          frame #4 {
            n772 = local write "Main Calibration Tab"(T7."Main" ("Main Calibration Tab")) -> ()
            n773 = local write "Tab Control 4"(T12."Main" ("Tab Control 4")) -> ()
          }
        }
      }
      event "TEMPERATURE STEP  Back 4", "TEMPERATURE STEP 1 Back 3", "TEMPERATURE STEP  Back 3", "TEMPERATURE STEP 1 Back 2", "Back Air TEMPERATURE Step 4", "Back SAMPLE TEMPERATURE Step 4": Value Change {
        # "Back Stroke step main temperature"
        n774 = event-data() -> ()  [unwired: 1 in, 6 out]
        n775 = stacked-sequence {
          frame #0 {
            n776 = Wait (ms)(milliseconds to wait=u32 1000) -> ()  [unwired: 1 out]
          }
          frame #1 {
            # "CAL;END"
            n777 = local write "Due Write"("CAL;END" ("Command")) -> ()
          }
          frame #2 {
            n778 = Wait (ms)(milliseconds to wait=u32 1000) -> ()  [unwired: 1 out]
          }
          frame #3 {
            # "CAL;END"
            n779 = local write "Due Write"("CAL;END" ("Command")) -> ()
          }
          frame #4 {
            # "TEMPERATURE STEP  Back 4"
            n780 = local write "Main Calibration Tab"(T7."Temperature" ("Main Calibration Tab")) -> ()
            n781 = local write "Tab Control 4"(T12."Main" ("Tab Control 4")) -> ()
          }
        }
      }
      event "FF BACK", "FF BACK 2", "FF BACK 3", "FF BACK 4", "FF BACK 5", "FF BACK 6": Value Change {
        n782 = event-data() -> ()  [unwired: 1 in, 6 out]
        n783 = stacked-sequence {
          frame #0 {
            n784 = Wait (ms)(milliseconds to wait=u32 1500) -> ()  [unwired: 1 out]
          }
          frame #1 {
            n785 = local write "Due Write"("VC;0") -> ()
          }
          frame #2 {
            n786 = Wait (ms)(milliseconds to wait=u32 1500) -> ()  [unwired: 1 out]
          }
          frame #3 {
            n787 = local write "Due Write"("VC;0") -> ()
          }
          frame #4 {
            w819 = FALSE
            n788 = local write "FF BACK 2"(w819) -> ()
            n789 = local write "FF BACK 3"(w819) -> ()
            n790 = local write "FF BACK 4"(w819) -> ()
            n791 = local write "FF BACK 5"(w819) -> ()
            n792 = local write "FF BACK 6"(w819) -> ()
            n793 = local write "FF BACK"(w819) -> ()
          }
          frame #5 {